vi "ZMQ publisher example.vi"() -> ()   [LabVIEW 2020]
uses:
  <vilib>/addons/zeromq/socket_type.ctl
  <vilib>/addons/zeromq/zeromq.lvlib
  <vilib>/addons/zeromq/zmq_context.lvclass
  <vilib>/addons/zeromq/zmq_socket.lvclass
panel:
  out "save time 2":u32(graph)
  in  "imput string":string
  out "error out":errorcluster
  out "string flatten time":u32
  in  "Stop":bool
  out "message":string[](array[string])
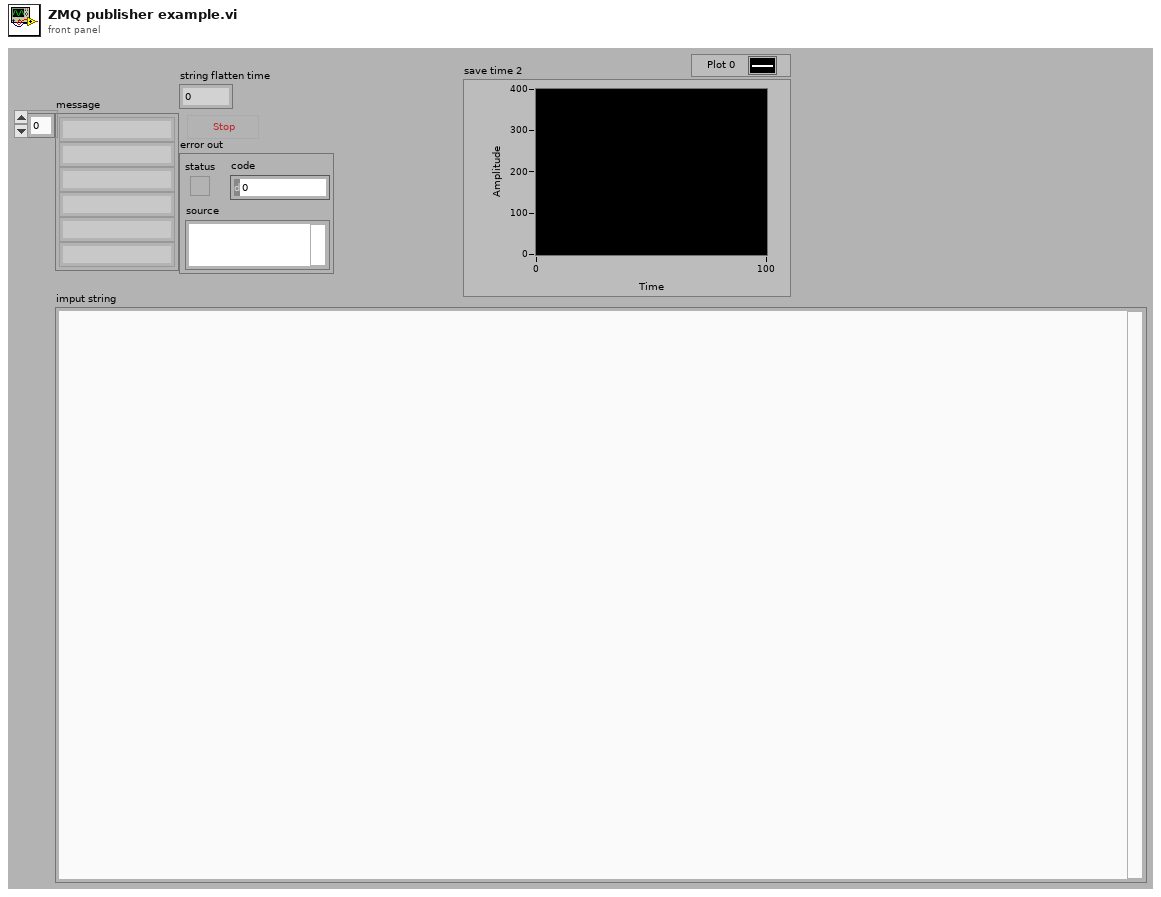
[diagram p1: front panel]
types:
  T1 = typedef "zeromq.lvlib/socket_type.ctl" = enum8{"ZMQ_PAIR", "ZMQ_PUB", "ZMQ_SUB", "ZMQ_REQ", "ZMQ_REP", "ZMQ_DEALER", "ZMQ_ROUTER", "ZMQ_PULL", "ZMQ_PUSH", "ZMQ_XPUB", "ZMQ_XSUB", "ZMQ_STREAM", "ZMQ_SERVER", "ZMQ_CLIENT", "ZMQ_RADIO", "ZMQ_DISH", "ZMQ_GATHER", "ZMQ_SCATTER", "ZMQ_DGRAM"}
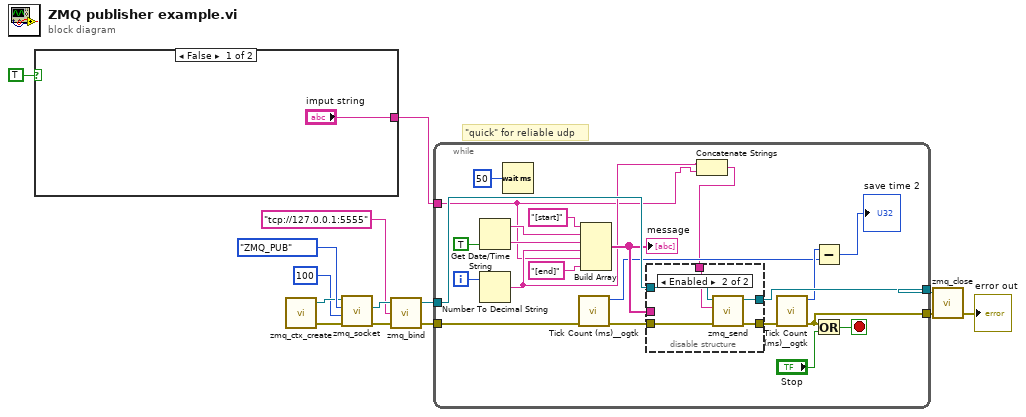
[diagram p0: block diagram]
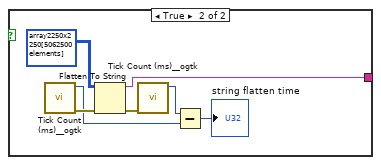
[diagram p2: hidden frame]
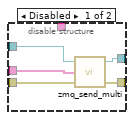
[diagram p3: hidden frame]
diagram:
  # "\"quick\" for reliable udp"
  n1 = case shown="False" TRUE {
    tunnel: ["imput string" w21] -> w6
    frame False {
    }
    frame True {
      n2 = call <userlib>:"Tick Count (ms)__ogtk.vi"() -> ("error out"=w20:errorcluster, "millisecond timer value"=w17:u32)  [unwired: 10 in]
      n3 = Flatten To String(anything=u16[][] array2250x2250[5062500 elements] ("Array"), error in (no error)=w20) -> (data string=w21:string, error out=w19:errorcluster)  [unwired: 2 in, 1 out]
      n4 = call <userlib>:"Tick Count (ms)__ogtk.vi"("error in (no error)"=w19) -> ("millisecond timer value"=w18:u32)  [unwired: 9 in, 1 out]
      n5 = Subtract(x=w18, y=w17) -> (x-y=→"string flatten time":u32)
    }
  }
  n6 = call <vilib>:"zmq_ctx_create.vi"() -> ("error out"=w12:errorcluster, "context out"=w9:refnum<class "zmq_context.lvclass">)  [unwired: 4 in]
  n7 = call <vilib>:"zmq_socket.vi"("error in"=w12, "linger (ms)"=100, "socket type"=socket_type."ZMQ_PUB", "context in"=w9) -> ("error out"=w11:errorcluster, "socket out"=w8:refnum<class "zmq_socket.lvclass">)  [unwired: 1 in, 1 out]
  n8 = call <vilib>:"zmq_bind.vi"("error in"=w11, "endpoint"="tcp://127.0.0.1:5555", "socket in"=w8) -> ("error out"=w10:errorcluster, "socket out"=w14:refnum<class "zmq_socket.lvclass">)  [unwired: 1 in]
  n9 = while {
    tunnel: w14 -> [w43]
    tunnel: w10 -> [w31]
    tunnel: w6 -> [w24]
    tunnel: [w33] -> w3
    tunnel: [w29] -> w2
    i -> [w38]
    stop <- w36 stop-if-true
    n10 = Get Date/Time String(want seconds? (F)=TRUE) -> (date string=w42:string, time string=w41:string)  [unwired: 2 in]
    n11 = Number To Decimal String(number=w38) -> (decimal integer string=w25:string)  [unwired: 1 in]
    n12 = Wait (ms)(milliseconds to wait=u32 50) -> ()  [unwired: 1 out]
    n13 = call <userlib>:"Tick Count (ms)__ogtk.vi"("error in (no error)"=w31) -> ("error out"=w32:errorcluster, "millisecond timer value"=w27:u32)  [unwired: 9 in]
    n14 = Build Array("[start]" ("element"), w42, w41, w25, w24, "[end]" ("element")) -> (w34:string[])
    "message" <- w34
    n15 = Concatenate Strings(w25, w24) -> (w23:string)
    n16 = disable-structure shown="Enabled" {
      disable-tunnel: w43 -> [w49 w54]
      disable-tunnel: w32 -> [w48 w52]
      disable-tunnel: [w47 w51] -> w30
      disable-tunnel: w34 -> [w46 _]
      disable-tunnel: w23 -> [_ w53]
      disable-tunnel: [w45 w50] -> w33
      frame Disabled {
        n17 = call <vilib>:"zmq_send_multi.vi"("error in"=w48, "parts"=w46, "socket in"=w49) -> ("error out"=w47:errorcluster, "socket out"=w45:refnum<class "zmq_socket.lvclass">)  [unwired: 1 in]
      }
      frame Enabled {
        n18 = call <vilib>:"zmq_send.vi"("error in"=w52, "data"=w53, "socket in"=w54) -> ("error out"=w51:errorcluster, "socket out"=w50:refnum<class "zmq_socket.lvclass">)  [unwired: 4 in]
      }
    }
    n19 = call <userlib>:"Tick Count (ms)__ogtk.vi"("error in (no error)"=w30) -> ("error out"=w29:errorcluster, "millisecond timer value"=w28:u32)  [unwired: 9 in]
    n20 = Subtract(x=w28, y=w27) -> (x-y=→"save time 2":u32)
    n21 = Or(x=w29, y="Stop") -> (x .or. y?=w36:bool)
  }
  n22 = call <vilib>:"zmq_close.vi"("error in"=w2, "socket"=w3) -> ("error out"=→"error out":errorcluster)  [unwired: 3 in]
